vi "inject curve on intensity plot.vi"(5 "graph para":T1={"x offset"=-10.0, "y offset"=0.0, "x scale"=0.1, "y scale"=0.002}, 7 "diff para":T2={"x0"=-1.0, "Ic0"=2.0, "h0"=1.0, "y0"=0.0}, 11 "IV Intensity":dbl[][](array[numeric])=array201x1000[201000 elements]) -> (3 "IV Intensity 2":dbl[][](graph))   [LabVIEW 2024]
uses:
  diff para.ctl
  graph para.ctl
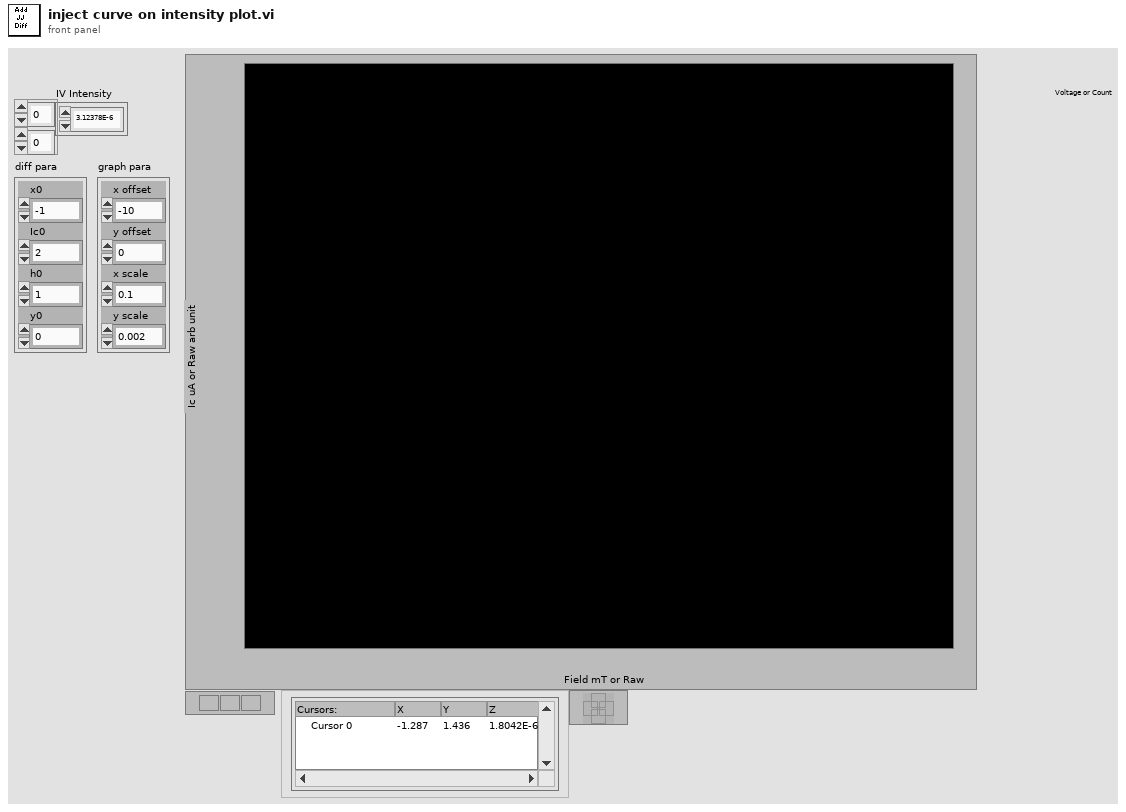
[diagram p1: front panel]
types:
  T1 = typedef "graph para.ctl" = cluster{"x offset":dbl, "y offset":dbl, "x scale":dbl, "y scale":dbl}
  T2 = typedef "diff para.ctl" = cluster{"x0":dbl, "Ic0":dbl, "h0":dbl, "y0":dbl}
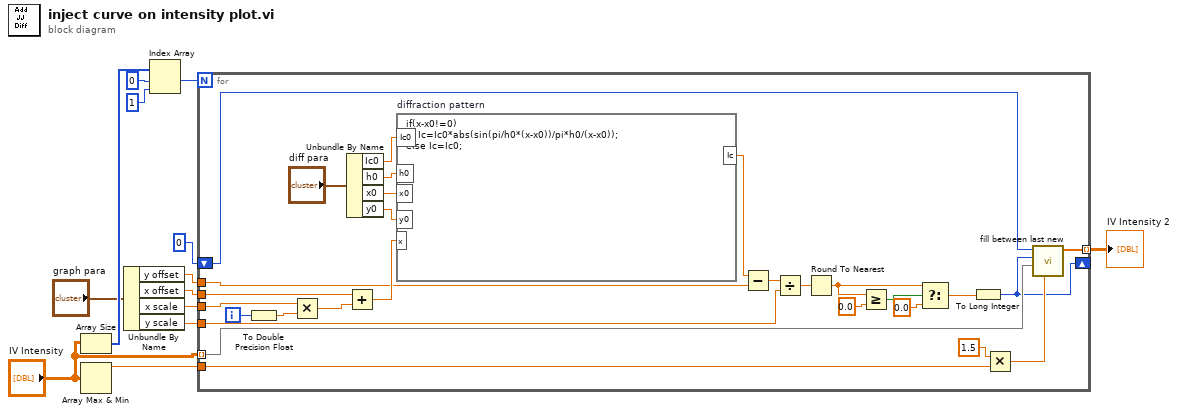
[diagram p0: block diagram]
diagram:
  n1 = Array Size(array="IV Intensity") -> (size(s)=w13:i32[])
  n2 = Array Max & Min(array="IV Intensity") -> (max value=w8:dbl)  [unwired: 3 out]
  n3 = Unbundle By Name("graph para") -> ("y offset"=w4:dbl, "x offset"=w3:dbl, "x scale"=w2:dbl, "y scale"=w1:dbl)
  n4 = Index Array(array=w13, index #1=0 ("index"), index #2=1 ("index")) -> (element #1=w10:i32)  [unwired: 1 out]
  n5 = for {
    N: w10 -> [_]
    tunnel: w2 -> [w40]
    tunnel: w3 -> [w37]
    tunnel: w4 -> [w34]
    tunnel: w1 -> [w32]
    tunnel: "IV Intensity" -> [w25] mode=indexing
    tunnel: w8 -> [w24]
    tunnel: [w23] -> w7 mode=indexing
    shift-right: [w21] -> _
    shift-left: 0 -> [w20]
    i -> [w41]
    n6 = To Double Precision Float(number=w41) -> (double precision float=w39:dbl)
    n7 = Multiply(x=w40, y=w39) -> (x*y=w38:dbl)
    n8 = Unbundle By Name("diff para") -> ("Ic0"=w17:dbl, "h0"=w16:dbl, "x0"=w15:dbl, "y0"=w14:dbl)
    n9 = Add(x=w37, y=w38) -> (x+y=w36:dbl)
    n10 = formula code="if(x-x0!=0)\n    Ic=Ic0*abs(sin(pi/h0*(x-x0))/pi*h0/(x-x0));\nelse Ic=Ic0;" "diffraction pattern"("Ic0"=w17, "h0"=w16, "x0"=w15, "y0"=w14, "x"=w36) -> ("Ic"=w35:dbl)
    n11 = Subtract(x=w35, y=w34) -> (x-y=w33:dbl)
    n12 = Divide(x=w33, y=w32) -> (x/y=w31:dbl)
    n13 = Round To Nearest(number=w31) -> (nearest integer value=w28:dbl)
    n14 = Greater Or Equal?(x=w28, y=0.0) -> (x >= y?=w29:bool)
    n15 = Select(t=w28, s=w29, f=0.0) -> (s? t:f=w26:dbl)
    n16 = To Long Integer(number=w26) -> (32bit integer=w21:i32)
    n17 = Multiply(x=1.5, y=w24) -> (x*y=w22:dbl)
    n18 = call "fill between last new.vi"("value"=w22, "array in"=w25, "New"=w21, "Last"=w20) -> ("array out"=w23:dbl[])  [unwired: 7 in]
  }
  "IV Intensity 2" <- w7
